vi "Main.vi"() -> ()   [LabVIEW 2020]
uses:
  System.Windows.Forms
  Global_Variable/Global.vi
  Global_Variable/A180648.vi
  <userlib>/_MGI/Menu Building/MenuTypes/MenuStrip/MGI_MenuStrip.lvclass
  <userlib>/_MGI/Menu Building/MenuItemStatusChange/MGI_MenuItemStatusChange.lvclass
  Libraries/S7/S7.lvlib
panel:
  out "状态":string
  out "客户软件版本号":string
  in  "Andon":enum32{"未选择", "缺料报警", "质量报警", "故障报警"}(radio)
  out "PLC":bool
  in  "菜单":refnum<k24>(container)
  in  "Result":string[][](table)
  out "逆向空载":bool
  out "试验计时":u16
  out "产品编号":string
  out "生产数量":i32
  out "合格数量":i32
  out "userStatus":string caption="用户状态"
  out "userName":string caption="用户名"
  out "connectionMode":string caption="联机类型"
  out "产品型号":string
  out "卡簧检测":bool
  out "拉力曲线":bool
  out "振动NVH":bool
  out "磨合":bool
  out "备用试验2":bool
  out "传感器特性":bool
  out "电流特性":bool
  out "端铆":bool
  in  "更换产品":refnum<vi>
  out "提示信息":string
  out "错误":bool
  out "时间字符串":string
  out "日期字符串":string
  out "自动":bool=TRUE
  # "上管柱上转向轴合成"
  # "试验项目"
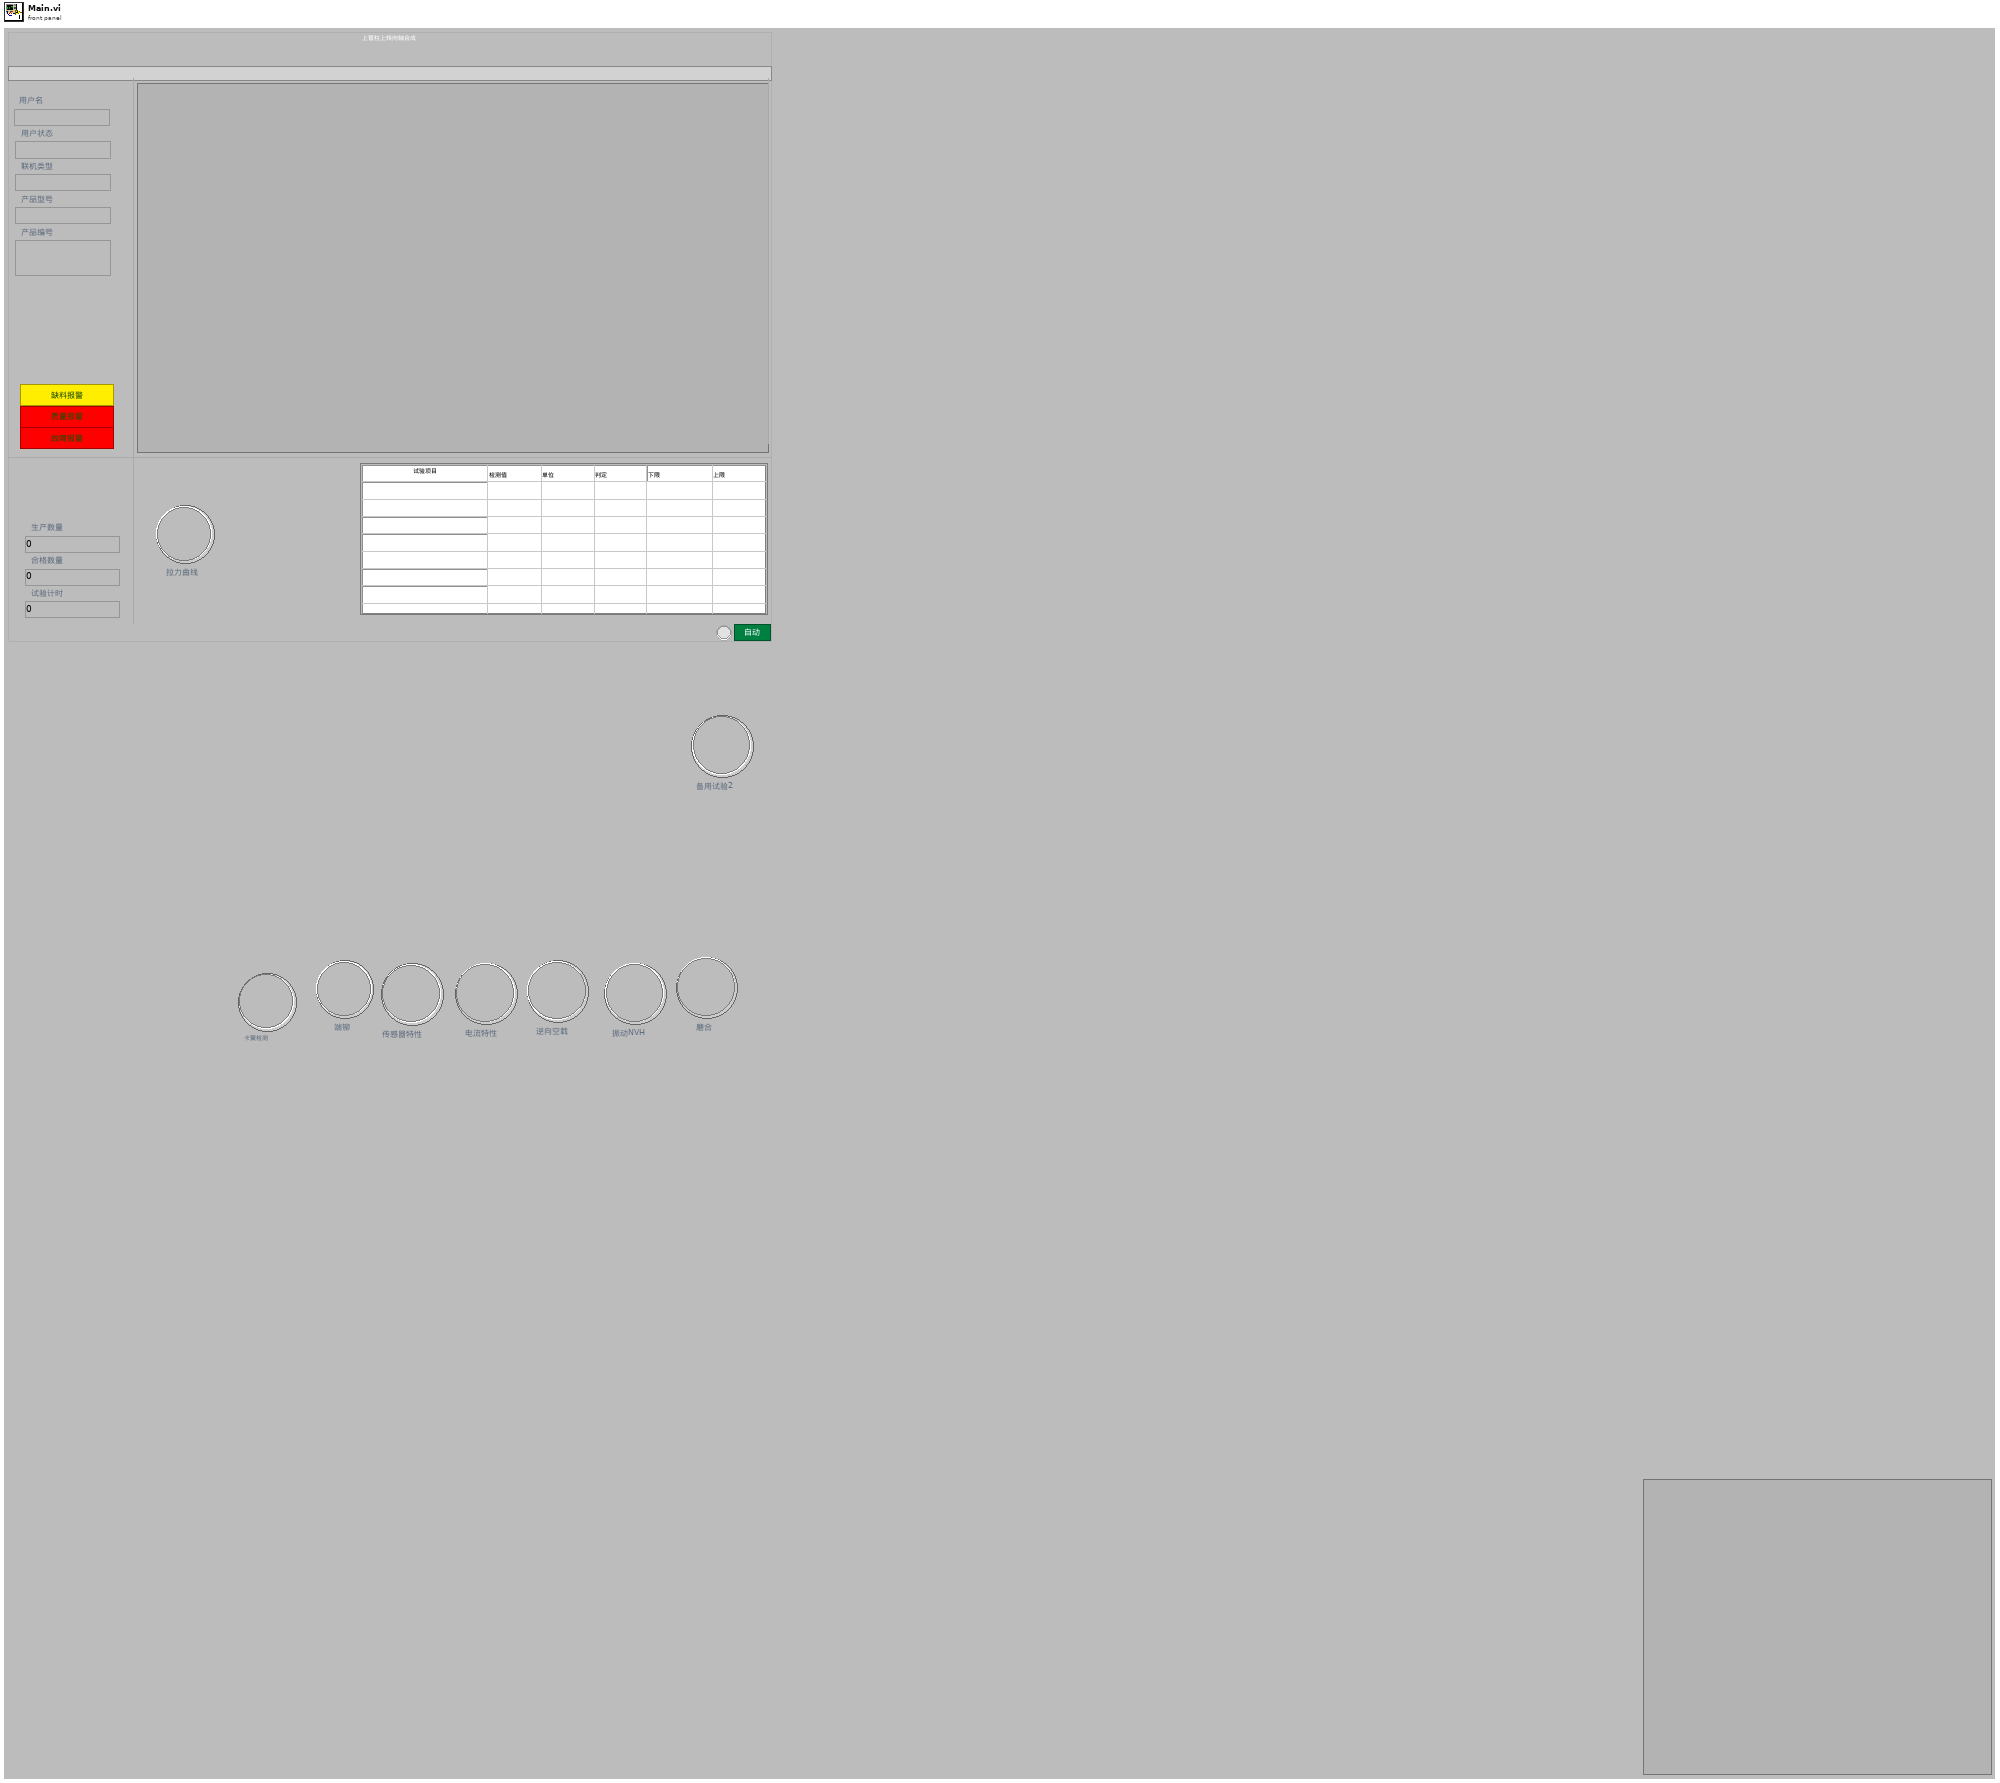
[diagram p1: front panel]
types:
  T1 = typedef "S7.lvlib/Broadcast Events--cluster.ctl" = cluster{"Module Did Init":refnum<user-event>, "Status Updated":refnum<user-event>, "Error Reported":refnum<user-event>, "Module Did Stop":refnum<user-event>, "Update Module Execution Status":refnum<user-event>}
  T2 = enum32{"轴承压装", "侧铆", "端铆", "力特性", "电流特性", "传感器特性", "逆向空载", "磨合"}
  T3 = enum32{"空载", "功能", "力特性", "电流特性", "传感器特性", "逆向空载", "磨合", "振动NVH"}
  T4 = enum32{"Invalid", "Standard", "Closed", "Hidden", "Minimized", "Maximized"}
  T5 = cluster{"设备名称":string, "操作人员":string, "设备状态":enum16{"设备离线", "设备正常", "设备缺料", "设备故障", "质量报警"}, "附加信息":string}
  T6 = enum32{"invalid app kind", "Development System", "Run Time System", "Student Edition", "Embedded LabVIEW", "Evaluation", "Custom"}
  T7 = cluster{"操作员编号":string, "操作员姓名":string, "操作员权限":string, "联机模式":enum16{"单机", "追溯"}}
  T8 = cluster{"Core":cluster{"Current VI Reference":refnum<vi>, "Close Panel on Exit?":bool}, "Your Boolean data":bool, "Your string data":string}
  T9 = cluster{"Current VI Reference":refnum<vi>, "Close Panel on Exit?":bool}
  T10 = cluster{"用户编号":string, "用户名":string, "用户密码(密文)":string, "用户权限":string}
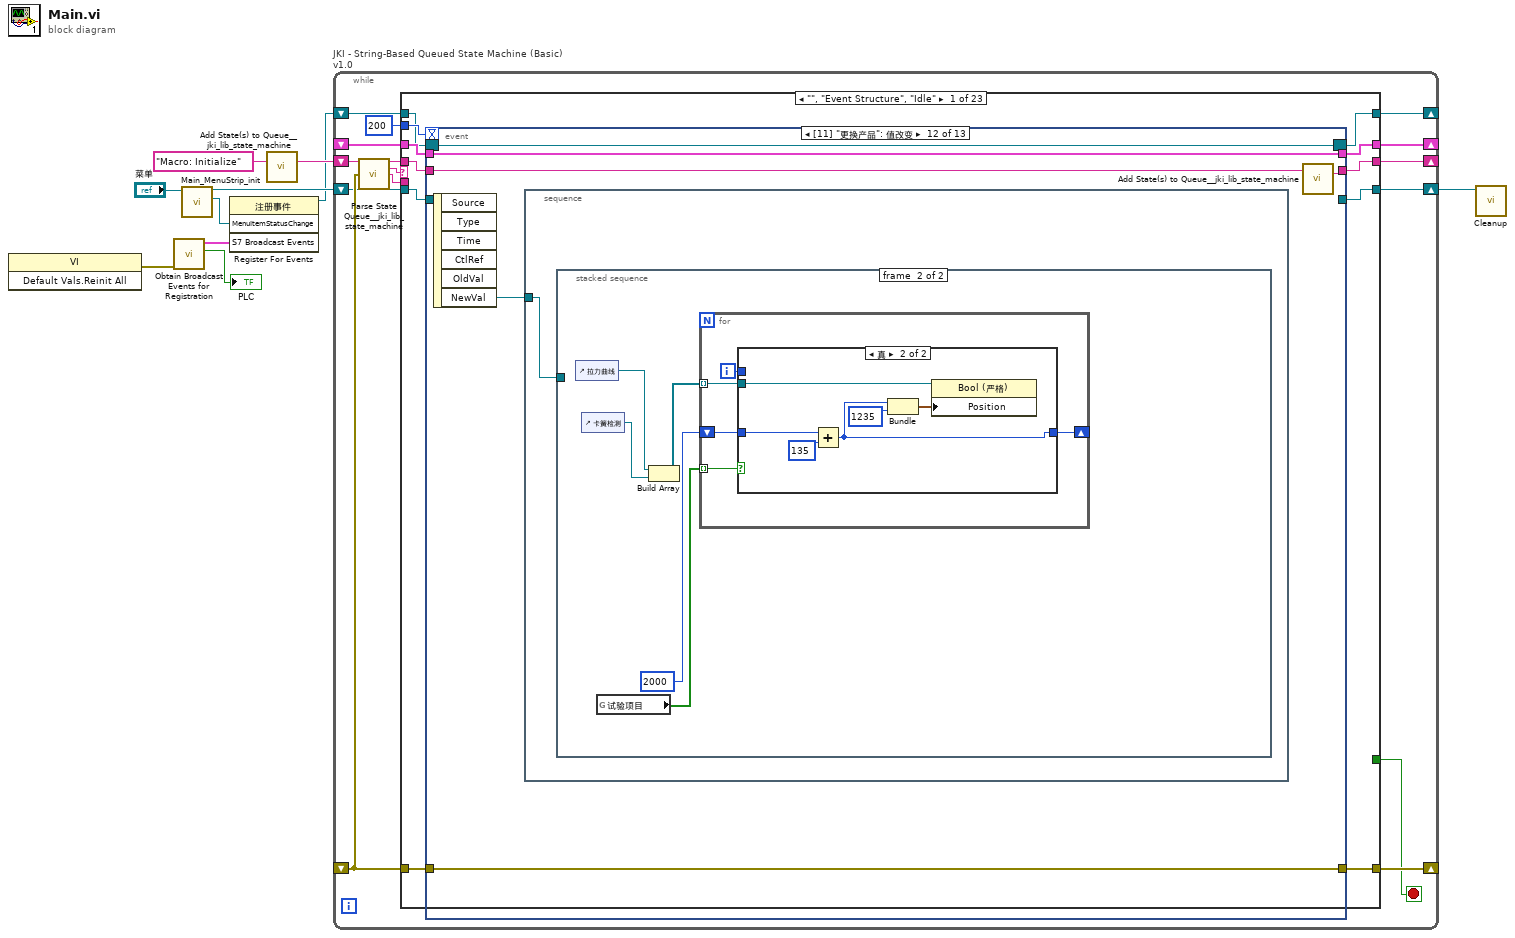
[diagram p0: block diagram]
diagram:
  n1 = invoke class="VI" method="Default Vals.Reinit All"() -> (error out=w3:errorcluster)  [unwired: 3 in, 2 out]
  n2 = call "Obtain Broadcast Events for Registration.vi"("error in (no error)"=w3) -> ("Already running?"=→"PLC":bool, "S7 Broadcast Events"=w5:T1)  [unwired: 8 in, 1 out]
  n3 = call "Main_MenuStrip_init.vi"("MenuStrip"="菜单") -> ("MenuItemStatusChange"=w2:refnum<user-event>, "Menu out"=w7:refnum<class "MGI_MenuStrip.lvclass">)  [unwired: 9 in]
  n4 = register-events(w2, w5) -> (reference out=w1:refnum<event-registration>)  [unwired: 2 in, 1 out]
  n5 = call <vilib>:"Add State(s) to Queue__jki_lib_state_machine.vi"("State(s) in (\"\")"="Macro: Initialize") -> ("States Out"=w10:string)  [unwired: 14 in]
  n6 = while "JKI - String-Based Queued State Machine (Basic) v1.0" {
    shift-right: [w19] -> _
    shift-left: _ -> [w18]
    shift-right: [w21] -> _
    shift-left: _ -> [w16]
    shift-right: [w20] -> _
    shift-left: w10 -> [w22]
    shift-right: [w14] -> w6
    shift-left: w7 -> [w15]
    shift-right: [w12] -> _
    shift-left: w1 -> [w11]
    stop <- w13 stop-if-true
    n7 = call <vilib>:"Parse State Queue__jki_lib_state_machine.vi"("State Queue"=w22, "Error In (no error)"=w16) -> ("Remaining States"=w24:string, "Current State"=w25:string, "Arguments"=w23:string)  [unwired: 11 in]
    n8 = case shown="\"\", \"Event Structure\", \"Idle\"" w25 {
      selector: w25 -> [_ _ w277 _ _ _ _ _ _ _ _ _ _ _ _ _ _ _ _ _ _ _ _]
      tunnel: w24 -> [w36 w274 w281 w301 w309 w316 w322 w326 w332 w338 w344 w353 w364 w372 w378 w385 w399 w435 w443 w456 w484 w491 w503]
      tunnel: w23 -> [_ _ _ _ _ _ _ _ _ _ _ _ _ _ _ _ _ _ w438 w450 _ _ _]
      tunnel: w18 -> [w34 w271 w279 w292 w306 w314 w319 w327 w335 w341 w347 w350 _ w367 w375 w383 w397 w432 w441 w452 w481 w488 w500]
      tunnel: [w33 w272 w283 w298 errorcluster {"status"=FALSE, "code"=0, "source"=""} ("error out") w313 w320 w324 w330 w337 w343 w351 w361 w368 w376 w382 w395 w433 w439 w453 w482 w489 w501] -> w21
      tunnel: w16 -> [w32 w272 w282 w298 w305 w313 w320 w324 w331 w337 w343 w351 w361 w369 w376 w379 w395 w433 w440 w454 w482 w489 w501]
      tunnel: [w35 w273 w280 w300 w308 w315 w321 w326 w333 w339 w345 w352 w363 w371 w377 w384 w398 w434 w442 w455 w483 w490 w502] -> w20
      tunnel: [w31 w271 w279 w299 w306 w314 w319 w327 w335 w341 w347 w350 w362 w367 w375 w383 w397 w432 w441 w452 w481 w488 w500] -> w19
      tunnel: 200 ("Timeout") -> [w30 _ _ _ _ _ _ _ _ _ _ _ _ _ _ _ _ _ _ _ _ _ _]
      tunnel: w15 -> [w29 w270 w276 w289 w303 w312 w318 w325 w334 w340 w346 w349 w355 w366 w374 w381 w396 w431 w437 w449 w480 w486 w493]
      tunnel: [w28 w270 w276 w289 w303 w312 w318 w325 w334 w340 w346 w349 w355 w366 w374 w381 w396 w431 w437 w449 w480 w486 w493] -> w14
      tunnel: [_ _ _ _ _ TRUE _ _ _ _ _ _ _ _ _ _ _ _ _ _ _ _ _] -> w13
      tunnel: [w26 w269 w275 w288 w302 w310 w317 w328 w329 w336 w342 w348 w356 w365 w373 w380 w394 w428 w436 w448 w479 w485 w492] -> w12
      tunnel: w11 -> [w27 w269 w275 w288 w302 w310 w317 w328 w329 w336 w342 w348 w356 w365 w373 w380 w394 w428 w436 w448 w479 w485 w492]
      frame "", "Event Structure", "Idle" {
        n9 = event shown="[11] \"更换产品\": 值改变" {
          selector: w27 -> [w39 w64 w86 w92 w158 w165 w172 w179 w193 w205 w212 w220 _]
          dyn-events: [w39 w64 w85 w92 w158 w165 w172 w179 w193 w205 w212 w220 _] -> w26
          timeout: w30 -> [_ _ _ _ _ _ _ _ _ _ _ _ _]
          tunnel: w36 -> [w51 w67 w90 w101 w159 w166 w175 w182 w190 w209 w219 w222 w263]
          tunnel: [w50 w66 w90 w99 w160 w167 w176 w183 w191 w210 w218 w223 w263] -> w35
          tunnel: w34 -> [w49 w68 w91 w100 w162 w170 w177 w184 w192 w211 w216 w225 w264]
          tunnel: [w40 w65 w87 w102 w163 w168 w173 w185 w188 w208 w217 w224 w261] -> w33
          tunnel: w32 -> [w40 w65 w88 w102 w163 w168 w173 w186 w188 w208 w217 w224 w261]
          tunnel: [w49 w68 w91 w100 w162 w170 w177 w184 w192 w211 w216 w225 w264] -> w31
          tunnel: w29 -> [w38 _ w89 w95 w161 w169 w174 w181 w189 _ _ _ w262]
          tunnel: [w38 _ w89 w95 w161 w169 w174 w181 w189 _ _ _ w262] -> w28
          event Timeout {
            n10 = event-data() -> ()  [unwired: 1 in, 1 out]
            n11 = global read "Global.vi" "计时开始"() -> (w42:bool)
            n12 = global read "Global.vi" "软件版本号"() -> (→"客户软件版本号":string)
            n13 = case shown="真" w42 {
              frame False {
                n14 = global write "Global.vi" "计时复位"(TRUE ("计时复位")) -> ()
              }
              frame True {
                n15 = stacked-sequence {
                  frame #0 {
                    n16 = global read "Global.vi" "计时复位"() -> (w53:bool)
                    n17 = call "已用时间"("Reset"=w53) -> ("Elapsed Time (s)"=→"试验计时":dbl)  [unwired: 11 in, 7 out]
                  }
                  frame #1 {
                    n18 = global write "Global.vi" "计时复位"(FALSE ("计时复位")) -> ()
                  }
                }
              }
            }
            n19 = Format Date/Time String(time format string (%c)="%H:%M ") -> (date/time string=→"时间字符串":string)  [unwired: 2 in]
            n20 = Format Date/Time String(time format string (%c)="%Y年%m月%d日") -> (date/time string=→"日期字符串":string)  [unwired: 2 in]
            n21 = call <vilib>:"Add State(s) to Queue__jki_lib_state_machine.vi"("State(s) in (\"\")"=w51) -> ("States Out"=w50:string)  [unwired: 14 in]
            n22 = global read "Global.vi" "合格数量"() -> (→"合格数量":i32)
            n23 = global read "Global.vi" "生产数量"() -> (→"生产数量":i32)
            n24 = global read "Global.vi" "产品编号"() -> (→"产品编号":string)
          }
          event "拉力曲线", "卡簧检测", "端铆", "传感器特性", "电流特性", "振动NVH", "逆向空载", "磨合": Mouse Down {
            w57 = refnum<user-event> refnum items=["轴承压装", "侧铆", "端铆", "力特性", "电流特性", "传感器特性", "逆向空载", "磨合"] ("用户事件输出")
            n25 = event-data() -> ("CtlRef"=w61:refnum<vi>)  [unwired: 1 in]
            n26 = property class="Bool (严格)"(reference=w61) -> ("Label.Text"=w60:string)  [unwired: 1 in, 2 out]
            n27 = vi-ref "Auto.vi"() -> (w63:refnum<vi>)
            n28 = case shown="\"侧铆\"" w60 {
              tunnel: [T2."轴承压装" ("试验项目") T2."侧铆" ("试验项目") T2."端铆" ("试验项目") T3."传感器特性" ("事件数据") T3."电流特性" ("事件数据") T3."逆向空载" ("事件数据") T3."振动NVH" ("事件数据") T3."磨合" ("事件数据")] -> w59
              frame "拉力曲线", Default {
              }
              frame "侧铆" {
              }
              frame "端铆" {
              }
              frame "传感器特性" {
              }
              frame "电流特性" {
              }
              frame "逆向空载" {
              }
              frame "振动NVH" {
              }
              frame "磨合" {
              }
            }
            n29 = invoke class="VI" method="Ctrl Val.Get"(reference=w63, "Control Name"="用户事件输出" ("控件名")) -> ("Get Control Value Variant"=w62:variant)  [unwired: 2 in, 3 out]
            n30 = Variant To Data(type=w57, Variant=w62) -> (data=w56:refnum<user-event>)  [unwired: 1 in, 1 out]
            n31 = Generate User Event(user event=w56, event data cluster=w59) -> ()  [unwired: 2 in, 2 out]
            n32 = call <vilib>:"Add State(s) to Queue__jki_lib_state_machine.vi"("State(s) in (\"\")"=w67) -> ("States Out"=w66:string)  [unwired: 14 in]
          }
          event "PLC": Value Change; "PLC": Mouse Down {
            # "141"
            n33 = event-data() -> ()  [unwired: 1 in, 4 out]
            n34 = call "Start Module.vi"("error in (no error)"=w88) -> ("error out"=w79:errorcluster, "Wait for Event Sync?"=w84:bool, "S7 Broadcast Events"=w83:T1, "Module Was Already Running?"=w82:bool)  [unwired: 7 in]
            n35 = local write "PLC"(w82) -> ()
            n36 = register-events(reference=w86, error in=w79, w83) -> (reference out=w85:refnum<event-registration>, error out=w78:errorcluster)  [unwired: 1 in]
            n37 = call "Synchronize Module Events.vi"("error in (no error)"=w78, "Wait for Event Sync?"=w84) -> ("error out"=w77:errorcluster)  [unwired: 9 in]
            n38 = call "Init S7 Link.vi"("error in (no error)"=w77, "超时"=500, "IP"="192.168.0.161") -> ("error out"=w87:errorcluster)  [unwired: 8 in]
          }
          event User Event {
            n39 = event-data() -> ("StatusChange"=w93:refnum<class "MGI_MenuItemStatusChange.lvclass">)  [unwired: 1 in]
            n40 = call <userlib>:"BasicInfo.vi"("MGI_MenuItemStatusChange in"=w93) -> ("Enabled?"=w96:bool, "Checked?"=w97:bool, "Tag"=w98:string)  [unwired: 7 in, 1 out]
            n41 = case shown="\"退出\"" w98 {
              tunnel: w97 -> [_ _ _ _ _ _ _ _ _ _ _ _ _ _ _]
              tunnel: w96 -> [_ _ _ _ _ _ _ _ _ _ _ _ _ _ _]
              tunnel: [_ _ "S7: Stop\nMacro: Exit" _ _ _ _ _ _ _ _ _ _ _ _] -> w94
              frame "假", Default {
              }
              frame "数据库配置" {
                n42 = global read "用户信息.vi" "用户信息"() -> (w104:T7)
                n43 = Unbundle By Name(w104) -> ("操作员权限"=w103:string)
                n44 = case shown="\"系统管理员\"" w103 {
                  frame Default {
                    n45 = One Button Dialog(message="权限不足！" ("消息")) -> ()  [unwired: 1 in, 1 out]
                  }
                  frame "系统管理员" {
                    n46 = vi-ref "数据库配置.vi"() -> (w107:refnum<vi>)
                    n47 = call "CallVI.vi"("VI引用"=w107, "状态"=T4."Standard") -> ()  [unwired: 12 in, 2 out]
                  }
                }
              }
              frame "退出" {
                n48 = global write "Global.vi" "程序关闭"(TRUE ("程序关闭")) -> ()
                n49 = call "Close_Client.vi"() -> ()  [unwired: 12 in]
              }
              frame "手动控制" {
                n50 = global read "用户信息.vi" "用户信息"() -> (w111:T7)
                n51 = Unbundle By Name(w111) -> ("操作员权限"=w110:string)
                n52 = case shown="\"班组长\", \"系统管理员\"" w110 {
                  frame Default {
                    n53 = One Button Dialog(message="权限不足！" ("消息")) -> ()  [unwired: 1 in, 1 out]
                  }
                  frame "班组长", "系统管理员" {
                    n54 = vi-ref "IO.vi"() -> (w114:refnum<vi>)
                    n55 = call "CallVI.vi"("VI引用"=w114, "状态"=T4."Standard") -> ()  [unwired: 12 in, 2 out]
                  }
                }
              }
              frame "半自动控制" {
                n56 = disable-structure shown="启用" {
                  frame Disabled {
                    n57 = shared-variable "我的电脑\\Global.lvlib\\操作者权限"() -> (w115:string)  [unwired: 1 in, 1 out]
                    n58 = case shown="\"班组长\", \"系统管理员\"" w115 {
                      frame Default {
                        n59 = One Button Dialog(message="权限不足！" ("消息")) -> ()  [unwired: 1 in, 1 out]
                      }
                      frame "班组长", "系统管理员" {
                        n60 = call "CallVI.vi"("VI引用"=refnum<vi> refnum, "状态"=T4."Maximized") -> ()  [unwired: 12 in, 2 out]
                      }
                    }
                  }
                  frame Enabled {
                    n61 = One Button Dialog(message="当前设备不具备半自动功能！" ("消息")) -> ()  [unwired: 1 in, 1 out]
                  }
                }
              }
              frame "产品管理" {
                n62 = vi-ref "Config.vi"() -> (w121:refnum<vi>)
                n63 = call "CallVI.vi"("VI引用"=w121, "状态"=T4."Standard") -> ()  [unwired: 12 in, 2 out]
              }
              frame "系统配置" {
                n64 = global read "用户信息.vi" "用户信息"() -> (w123:T7)
                n65 = Unbundle By Name(w123) -> ("操作员权限"=w122:string)
                n66 = case shown="\"班组长\", \"系统管理员\"" w122 {
                  frame Default {
                    n67 = One Button Dialog(message="权限不足！" ("消息")) -> ()  [unwired: 1 in, 1 out]
                  }
                  frame "班组长", "系统管理员" {
                    n68 = vi-ref "Setting.vi"() -> (w126:refnum<vi>)
                    n69 = call "CallVI.vi"("VI引用"=w126, "状态"=T4."Standard") -> ()  [unwired: 12 in, 2 out]
                  }
                }
              }
              frame "用户管理" {
                n70 = global read "用户信息.vi" "用户信息"() -> (w128:T7)
                n71 = Unbundle By Name(w128) -> ("操作员权限"=w127:string)
                n72 = case shown="\"系统管理员\"" w127 {
                  frame Default {
                    n73 = One Button Dialog(message="权限不足！" ("消息")) -> ()  [unwired: 1 in, 1 out]
                  }
                  frame "系统管理员" {
                    n74 = vi-ref "User_manager.vi"() -> (w131:refnum<vi>)
                    n75 = call "CallVI.vi"("VI引用"=w131, "状态"=T4."Standard") -> ()  [unwired: 12 in, 2 out]
                  }
                }
              }
              frame "编码规则" {
                n76 = global read "用户信息.vi" "用户信息"() -> (w133:T7)
                n77 = Unbundle By Name(w133) -> ("操作员权限"=w132:string)
                n78 = case shown="\"班组长\", \"工艺管理员\", \"系统管理员\"" w132 {
                  frame Default {
                    n79 = One Button Dialog(message="权限不足！" ("消息")) -> ()  [unwired: 1 in, 1 out]
                  }
                  frame "班组长", "工艺管理员", "系统管理员" {
                    n80 = vi-ref "编码规则设置.vi"() -> (w136:refnum<vi>)
                    n81 = call "CallVI.vi"("VI引用"=w136, "状态"=T4."Standard") -> ()  [unwired: 12 in, 2 out]
                  }
                }
              }
              frame "易损件管理" {
                n82 = vi-ref "易损件管理.vi"() -> (w138:refnum<vi>)
                n83 = call "CallVI.vi"("VI引用"=w138, "状态"=T4."Standard") -> ()  [unwired: 12 in, 2 out]
              }
              frame "物料批次管理" {
                n84 = vi-ref "批次管理.vi"() -> (w140:refnum<vi>)
                n85 = call "CallVI.vi"("VI引用"=w140, "状态"=T4."Standard") -> ()  [unwired: 12 in, 2 out]
              }
              frame "报表" {
                n86 = call "文件对话框"("start path"=path "D:/report", "prompt"="打开报表", "pattern (all files)"="*.doc;*.docx", "pattern label"="Word 文档") -> ("selected path"=w141:path, "error out"=w142:errorcluster)  [unwired: 8 in, 2 out]
                n87 = case shown="无错误" w142 {
                  selector: w142 -> [w148 w150]
                  tunnel: w141 -> [w149 _]
                  frame No Error {
                    w147 = 1 items=["Normal", "Maximize", "Minimize"] ("cpubbs_WindowState")
                    n88 = call "Open_Word.vi"("File Path"=w149, "cpubbs_WindowState"=w147, "错误输入（无错误）"=w148) -> ()  [unwired: 12 in, 1 out]
                  }
                  frame Error {
                    n89 = call <vilib>:"Clear Errors.vi"("error in (no error)"=w150) -> ()  [unwired: 5 in, 2 out]
                  }
                }
              }
              frame "报警信息" {
                n90 = vi-ref "报警信息.vi"() -> (w152:refnum<vi>)
                n91 = call "CallVI.vi"("VI引用"=w152, "状态"=T4."Standard") -> ()  [unwired: 12 in, 2 out]
              }
              frame "关于" {
                n92 = vi-ref "About.vi"() -> (w154:refnum<vi>)
                n93 = call "CallVI.vi"("VI引用"=w154, "状态"=T4."Standard") -> ()  [unwired: 12 in, 2 out]
              }
              frame "操作演示" {
                n94 = call <vilib>:"Application Directory.vi"() -> ("Application Directory"=w157:path)
                n95 = Build Path(base path=w157, name or relative path="操作演示" ("名称或相对路径")) -> (appended path=w156:path)
                n96 = call "自动播放ppt.vi"("路径"=w156) -> ()  [unwired: 10 in, 1 out]
              }
            }
            n97 = call <vilib>:"Add State(s) to Queue__jki_lib_state_machine.vi"("State(s) in (\"\")"=w101, "State(s) at Back (\"\")"=w94) -> ("States Out"=w99:string)  [unwired: 13 in]
          }
          event User Event {
            n98 = event-data() -> ("Init?"=w164:bool)  [unwired: 1 in, 1 out]
            n99 = local write "PLC"(w164) -> ()
            n100 = call <vilib>:"Add State(s) to Queue__jki_lib_state_machine.vi"("State(s) in (\"\")"=w159) -> ("States Out"=w160:string)  [unwired: 14 in]
          }
          event User Event {
            n101 = event-data() -> ("Running?"=w171:bool)  [unwired: 1 in]
            n102 = local write "PLC"(w171) -> ()
            n103 = call <vilib>:"Add State(s) to Queue__jki_lib_state_machine.vi"("State(s) in (\"\")"=w166) -> ("States Out"=w167:string)  [unwired: 14 in]
          }
          event User Event {
            n104 = event-data() -> ()  [unwired: 1 in, 7 out]
            n105 = local write "PLC"(FALSE ("PLC")) -> ()
            n106 = call <vilib>:"Add State(s) to Queue__jki_lib_state_machine.vi"("State(s) in (\"\")"=w175) -> ("States Out"=w176:string)  [unwired: 14 in]
          }
          event User Event {
            n107 = event-data() -> ("Error"=w187:errorcluster)  [unwired: 1 in]
            n108 = Merge Errors(w187, w186) -> (w185:errorcluster)
            n109 = call <vilib>:"Add State(s) to Queue__jki_lib_state_machine.vi"("State(s) in Front (\"\")"="S7: Initialize\nIdle", "State(s) in (\"\")"=w182) -> ("States Out"=w183:string)  [unwired: 13 in]
          }
          event "自动": Mouse Down {
            n110 = event-data() -> ()  [unwired: 1 in, 1 out]
            n111 = disable-structure shown="禁用" {
              frame Disabled {
                n112 = local read "自动"() -> (w194:bool)
                n113 = case shown="真" w194 {
                  frame False {
                    n114 = call "设备状态.vi"() -> ("Status_Read"=w195:i16)  [unwired: 11 in]
                    n115 = case shown="5" w195 {
                      frame 0, Default {
                        n116 = One Button Dialog(message="请复位！" ("消息")) -> ()  [unwired: 1 in, 1 out]
                      }
                      frame 5 {
                        n117 = vi-ref "Auto.vi"() -> (w199:refnum<vi>)
                        n118 = invoke class="VI" method="Ctrl Val.Set"(reference=w199, "Control Name"="STEP" ("控件名"), "Value"="进入自动" ("控件名")) -> ()  [unwired: 2 in, 5 out]
                      }